vi "SMain.vi"() -> ()   [LabVIEW 2011]
uses:
  Data/ClassLibraryMisWebservice.dll
  dataType/informationIn.ctl
  dataType/singleTestParameter.ctl
  dataType/cluResult.ctl
  dataType/UploadPara.ctl
  Data/Interop.PLTS.dll
  <vilib>/Utility/NIReport.llb/NI_report.lvclass
  dataType/HW_xml.ctl
  Data/xmlFunction.dll
  <vilib>/Utility/file.llb/Read From Spreadsheet File (string).vi
  <vilib>/Utility/file.llb/Write To Spreadsheet File (string).vi
  <vilib>/addons/_office/excel.llb/Excel Easy Table (str).vi
  <vilib>/xml/Load XML File.vi
  <vilib>/regexp/Match Regular Expression.xnode
  <vilib>/Utility/NIReport.llb/Excel/NI_Excel.lvclass
  <vilib>/addons/_office/NI_ReportGenerationToolkit.lvlib
  <vilib>/xml/NI_XML.lvlib
panel:
  out "uploadPara":T1
  out "cluResult":T2
  out "FEXT Results":bool[](array[boolean])
  out "FEXTLIst":string[](array[string])
  out "NEXTList":string[](array[string])
  out "itemList":string[](array[string])
  out "sSpec":T3[](array[typedef])
  out "FEXT INF":T4={"Sample PN: "="", "SampleSN:"="", "Sparam Test Item"=[], "S-para Pair Name"=[], "Length"="", "Diff Test Item Name"=["SDD21", "SDD22", "SCD21", "SCD22", "SCC11", "NEXT", "FEXT"], "Diff Test Item Name smooth"=[], "smooth point"=0.0, "limitSpec"=[], "switchIndexOffset"=0.0, "testType"=enum."Loss"}
  out "NEXT INF":T4={"Sample PN: "="", "SampleSN:"="", "Sparam Test Item"=[], "S-para Pair Name"=[], "Length"="", "Diff Test Item Name"=["SDD21", "SDD22", "SCD21", "SCD22", "SCC11", "NEXT", "FEXT"], "Diff Test Item Name smooth"=[], "smooth point"=0.0, "limitSpec"=[], "switchIndexOffset"=0.0, "testType"=enum."Loss"}
  in  "Information In 2":T4={"Sample PN: "="", "SampleSN:"="", "Sparam Test Item"=[], "S-para Pair Name"=[], "Length"="", "Diff Test Item Name"=["SDD21", "SDD22", "SCD21", "SCD22", "SCC11", "NEXT", "FEXT"], "Diff Test Item Name smooth"=[], "smooth point"=0.0, "limitSpec"=[], "switchIndexOffset"=0.0, "testType"=enum."Loss"}
  out "limitSpec":string[][](array[string])
  in  "Information In":T4={"Sample PN: "="", "SampleSN:"="", "Sparam Test Item"=[], "S-para Pair Name"=[], "Length"="", "Diff Test Item Name"=["SDD21", "SDD22", "SCD21", "SCD22", "SCC11", "NEXT", "FEXT"], "Diff Test Item Name smooth"=[], "smooth point"=0.0, "limitSpec"=[], "switchIndexOffset"=0.0, "testType"=enum."Loss"}
  out "EEUPLOAD":bool
  out "caliData":string
  out "caliPassed":bool
  out "caliDataSelect":bool
  out "sampleData":string
  out "caliFlag":string="cali"
  in  "Stop":bool
  in  "IF Bandwidth:":enum16{"10KHz", "3KHz", "1KHz"}(ring)
  out "FixtureNo":string="111"
  out "LabelNum":i32
  in  "Project Name":u16(ring) items=["QSFP+_10G.xls", "QSFP+_IBM Project.xls"]
  out "S4P Data Path":path=path "D:/高频房软件/2. HPTS_VNA_Rev2.7.1.3-1107最新源码/Demo_data/THRU"
  out "boardCounts":string="Port0 Usage Frequency: 04\nPort1 Usage Frequency: 06" caption="BoardCounts"
  out "preStation":string
  out "original Path":path=path "D:/高频房软件/2. HPTS_VNA_Rev2.7.1.3-1107最新源码/Demo_data"
  in  "Test Spec":u16(ring) items=["EDR_Spec.xls", "QSFP+_10G_IBM.xls"]
  in  "End Page":i32=3
  in  "Start Page":i32=1
  in  "Compensation(ohm)":dbl
  in  "StopTimeNs":dbl=5.0
  in  "Data Points":i32=4000
  in  "Start TimeNs":dbl
  in  "Impedance Filter":bool=TRUE
  in  "Filter Risetime(ps)":dbl=30.0 min=1.0 max=1000.0 step=1.0
  in  "VNA Initial":bool caption="Start Test"
  out "EE Write":bool
  out "正常工单?":bool
  out "PN TYpe":string
  out "PN description":string
  out "NetLocalpath":string
  out "NetTemppath":string
  out "asychronus":bool
  out "show_Cable Point":dbl[](array[numeric])
  out "show_Terminal Point":dbl[](array[numeric])
  out "customerPN":string caption="删减后字符串"
  out "secondresult":bool[](array[boolean])
  out "usedSN":string
  out "Reference":T5
  out "TDR setting array":T6(array[cluster])
  out "CMP setting":string
  out "校验信息":T7(array[cluster])
  out "继续?":bool
  out "DB2":T8
  out "DB1":T8
  out "startSN":i32
  out "线别确认":bool
  out "测试模式":bool
  out "重测原因":string
  out "LastSN":string="automatic sn" caption="S/N:"
  out "TestResultSave":bool
  in  "TestResultSummary":T9={"auto get refer point"=FALSE, "width1"=0, "width2"=0, "show_TDD11"=[], "show_TDD22"=[], "test time"=["2016/11/14 11:59:03"], "show_impspec"=[], "TestResult"=[], "FileName"="", "FileVersion"=""}
  out "TestResult":bool[](array[boolean])
  in  "错误输入（无错误）":errorcluster
  out "2x equalize":bool
  out "Diff Test Item smooth":string[](array[string])=["SDD21", "SDD11,smooth", "SCD22", "SCC11", "SCD21-SDD21", "NEXT", "ILD_15"]
  out "smooth point":i32=5
  out "test result":bool
  out "TDR Setting 2":T10={"Start TimeNs"=0.0, "StopTimeNs"=5.0, "Data Points"=4000, "Compensation(ohm)"=0.0, "DataFormat"=6, "Impedance Filter"=TRUE, "Filter Risetime(ps)"=30.0, "Impedance Spec String"="0.75@110@2@110;0.75@90@2@95", "Skew Spec(ps)"=15, "CMP Setting"=""}
  in  "DataFormat":i16(ring)=6 items=["StepReal", "ImpulseReal", "StepVolts", "ImpulseVolts", "StepLog", "ImpulseLog", "StepImpedance"]
  out "Skew Spec(ps) 2":i32
  out "2X IL 2":dbl[](array[numeric])=[-0.025299, -0.038396, -0.047424, -0.055976, -0.059331, -0.068781, -0.07578, -0.081239, -0.089022, -0.093241, -0.097614, -0.102462, -0.106838, -0.111812, -0.116556, -0.121163, -0.12561, -0.131718, -0.134792, -0.13877, -0.145469, -0.149479, -0.152659, -0.157142, -0.162291, -0.164771, -0.168818, -0.17033, -0.176722, -0.179419, -0.183921, -0.186601, -0.190951, -0.193378, -0.19824, -0.20176, -0.202689, -0.207947, -0.211354, -0.214498, -0.220736, -0.223214, -0.225991, -0.227897, -0.231621, -0.235236, -0.238474, -0.242007, -0.244427, -0.24856, -0.251615, -0.255644, -0.257638, -0.261234, -0.264621, -0.266303, -0.269738, -0.272241, -0.274441, -0.276158, -0.279938, -0.282564, -0.28537, -0.288029, -0.292169, -0.294557, -0.297687, -0.301761, -0.304652, -0.305833, -0.307066, -0.309591, -0.312562, -0.315843, -0.31639, -0.31604, -0.318513, -0.320032, -0.322668, -0.32612, -0.330335, -0.334297, -0.34034, -0.341411, -0.345104, -0.347321, -0.349213, -0.351984, -0.354782, -0.356899, -0.357019, -0.361617, -0.362734, -0.36572, -0.367166, -0.371019, -0.372807, -0.37617, -0.378489, -0.380671, -0.383681, -0.385224, -0.386151, -0.388422, -0.389343, -0.39172, -0.393825, -0.397043, -0.398343, -0.400077, -0.405011, -0.406109, -0.409167, -0.410383, -0.411453, -0.41508, -0.417531, -0.419854, -0.421583, -0.424947, -0.42654, -0.429572, -0.430897, -0.434433, -0.435632, -0.438249, -0.440184, -0.442646, -0.444562, -0.445842, -0.447651, -0.450634, -0.452453, -0.454341, -0.457792, -0.459201, -0.460308, -0.461669, -0.462777, -0.464409, -0.468144, -0.470502, -0.47275, -0.475034, -0.475669, -0.478023, -0.478382, -0.480829, -0.482842, -0.484459, -0.486674, -0.489177, -0.491121, -0.494005, -0.495936, -0.497061, -0.499267, -0.50051, -0.502804, -0.50405, -0.505765, -0.507052, -0.509473, -0.512389, -0.51437, -0.515671, -0.517533, -0.519425, -0.52189, -0.521842, -0.52303, -0.525679, -0.528968, -0.530579, -0.532575, -0.53465, -0.536459, -0.537934, -0.539202, -0.54086, -0.542603, -0.5457, -0.547524, -0.548774, -0.549721, -0.552302, -0.554863, -0.556646, -0.559567, -0.560755, -0.564216, -0.565447, -0.56634, -0.567621, -0.568795, -0.572849, -0.573837, -0.573788, -0.575949, -0.580124, -0.580805, -0.583633, -0.584421, -0.586743, -0.588333, -0.590903, -0.592009, -0.594853, -0.595409, -0.597326, -0.596798, -0.597763, -0.60116, -0.60416, -0.606395, -0.609768, -0.610518, -0.612809, -0.614324, -0.616136, -0.617459, -0.618913, -0.618354, -0.620853, -0.624932, -0.626581, -0.630236, -0.632642, -0.633388, -0.63542, -0.635927, -0.636904, -0.638461, -0.640481, -0.642285, -0.643035, -0.645007, -0.647452, -0.650336, -0.650522, -0.650374, -0.652932, -0.654354, -0.6563, -0.657573, -0.660404, -0.661557, -0.664981, -0.665852, -0.666908, -0.670274, -0.671692, -0.672849, -0.675964, -0.679116, -0.680009, -0.680817, -0.682485, -0.684064, -0.685281, -0.685714, -0.689176, -0.689231, -0.691987, -0.693946, -0.696069, -0.697712, -0.700794, -0.701734, -0.703201, -0.703776, -0.705657, -0.708378, -0.71062, -0.711792, -0.713659, -0.715097, -0.716667, -0.718491, -0.720789, -0.721948, -0.722241, -0.724976, -0.726849, -0.72666, -0.729363, -0.730162, -0.732883, -0.735904, -0.736952, -0.739038, -0.73981, -0.741586, -0.743353, -0.745631, -0.747878, -0.748821, -0.750045, -0.751315, -0.75408, -0.756592, -0.758178, -0.759658, -0.76182, -0.762632, -0.764898, -0.765885, -0.768208, -0.769777, -0.771565, -0.77349, -0.77466, -0.77747, -0.77947, -0.780437, -0.783258, -0.784929, -0.787219, -0.78773, -0.789671, -0.791426, -0.793443, -0.795477, -0.798215, -0.798336, -0.800847, -0.801219, -0.804592, -0.804967, -0.807604, -0.808648, -0.811207, -0.812119, -0.814463, -0.816479, -0.816857, -0.818916, -0.820631, -0.82228, -0.824061, -0.826539, -0.829216, -0.830524, -0.832218, -0.833493, -0.834462, -0.836032, -0.838399, -0.839965, -0.843226, -0.842684, -0.844971, -0.848181, -0.849788, -0.85147, -0.853466, -0.8544, -0.856009, -0.85821, -0.860153, -0.862614, -0.863089, -0.865995, -0.866916, -0.869606, -0.87226, -0.872654, -0.873102, -0.874217, -0.875987, -0.878471, -0.880127, -0.881265, -0.883254, -0.885726, -0.887636, -0.888446, -0.889525, -0.89144, -0.89356, -0.895586, -0.89772, -0.898394, -0.901539, -0.902978, -0.903626, -0.905436, -0.907707, -0.908756, -0.91031, -0.911702, -0.913224, -0.914065, -0.915603, -0.917613, -0.918547, -0.920796, -0.921613, -0.925115, -0.926152, -0.927588, -0.930169, -0.931709, -0.932481, -0.934098, -0.936424, -0.936876, -0.937659, -0.939378, -0.941622, -0.943235, -0.942614, -0.945728, -0.946817, -0.949055, -0.95112, -0.95217, -0.955136, -0.957149, -0.957272, -0.959033, -0.9612, -0.961962, -0.963545, -0.967061, -0.968399, -0.970546, -0.973385, -0.973856, -0.974207, -0.975643, -0.97884, -0.97915, -0.980188, -0.982034, -0.98472, -0.986456, -0.988529, -0.989871, -0.992863, -0.994155, -0.996464, -0.998286, -0.999287, -1.000963, -1.001043, -1.002651, -1.00456, -1.007629, -1.008066, -1.009819, -1.01113, -1.013663, -1.014789, -1.017072, -1.019742, -1.021611, -1.023713, -1.025332, -1.026222, -1.026869, -1.027743, -1.030052, -1.03073, -1.033045, -1.035049, -1.036088, -1.03854, -1.041763, -1.042051, -1.043345, -1.044835, -1.045911, -1.047474, -1.050112, -1.050947, -1.054054, -1.056098, -1.056999, -1.058949, -1.060286, -1.061237, -1.061735, -1.064154, -1.066454, -1.068678, -1.068777, -1.071732, -1.07341, -1.073918, -1.07718, -1.078266, -1.080347, -1.081876, -1.083674, -1.084348, -1.085916, -1.086228, -1.089243, -1.090434, -1.091868, -1.094835, -1.096616, -1.096945, -1.099785, -1.102174, -1.103444, -1.10423, -1.105284, -1.106884, -1.107956, -1.108242, -1.110338, -1.113661, -1.114571, -1.117028, -1.118751, -1.119113, -1.121022, -1.123104, -1.122807, -1.125616, -1.127797, -1.12873, -1.12972, -1.132328, -1.133934, -1.136053, -1.13791, -1.138532, -1.139899, -1.141078, -1.142651, -1.141653, -1.145035, -1.146205, -1.147698, -1.149198, -1.151227, -1.15306, -1.155051, -1.157576, -1.158307, -1.160585, -1.161081, -1.162078, -1.164421, -1.165552, -1.167357, -1.16903, -1.16941, -1.172091, -1.173558, -1.175417, -1.177655, -1.179563, -1.180398, -1.181254, -1.183122, -1.184561, -1.185409, -1.186553, -1.188506, -1.190284, -1.19296, -1.194518, -1.196114, -1.199446, -1.199928, -1.201659, -1.203025, -1.204984, -1.205929, -1.207424, -1.20884, -1.212338, -1.213546, -1.216908, -1.219662, -1.222377, -1.223413, -1.224234, -1.224444, -1.226533, -1.227726, -1.229907, -1.230216, -1.233822, -1.235221, -1.23743, -1.238272, -1.239472, -1.240008, -1.241383, -1.242313, -1.244294, -1.245158, -1.247334, -1.248006, -1.250743, -1.251832, -1.252133, -1.253227, -1.255278, -1.256617, -1.257998, -1.258347, -1.259462, -1.262189, -1.26538, -1.265117, -1.267315, -1.267774, -1.269888, -1.271996, -1.272938, -1.272988, -1.276344, -1.278889, -1.280114, -1.282203, -1.282807, -1.2851, -1.286312, -1.28754, -1.289422, -1.290962, -1.293184, -1.295772, -1.297139, -1.300557, -1.30177, -1.303345, -1.303985, -1.306281, -1.307709, -1.309835, -1.309741, -1.312592, -1.315234, -1.317538, -1.319714, -1.322086, -1.323841, -1.32463, -1.326073, -1.327763, -1.329139, -1.329624, -1.331755, -1.332977, -1.33489, -1.33754, -1.339253, -1.342017, -1.344422, -1.345122, -1.345541, -1.346031, -1.346359, -1.3474, -1.348735, -1.349061, -1.350116, -1.353398, -1.354305, -1.357842, -1.356693, -1.358147, -1.359578, -1.360392, -1.361354, -1.363513, -1.364167, -1.365032, -1.366879, -1.367457, -1.368583, -1.370459, -1.371694, -1.373734, -1.376242, -1.379085, -1.379925, -1.379883, -1.381184, -1.381655, -1.38242, -1.38571, -1.387976, -1.390893, -1.394178, -1.396827, -1.399715, -1.402093, -1.404467, -1.404706, -1.405469, -1.407391, -1.409543, -1.41276, -1.414513, -1.419863, -1.421498, -1.423363, -1.425305, -1.426751, -1.426783, -1.428077, -1.428979, -1.43197, -1.434989, -1.437283, -1.438178, -1.440308, -1.441654, -1.442987, -1.443577, -1.44396, -1.443438, -1.445594, -1.44515, -1.445881, -1.448352, -1.449836, -1.450411, -1.451182, -1.452277, -1.453172, -1.453119, -1.453, -1.453989, -1.456489, -1.456532, -1.458466, -1.458938, -1.460769, -1.462027, -1.462978, -1.462454, -1.464558, -1.46441, -1.466658, -1.466867, -1.468869, -1.47093, -1.472731, -1.47355, -1.474344, -1.474451, -1.476897, -1.478554, -1.479486, -1.481271, -1.483897, -1.484711, -1.487268, -1.488311, -1.489221, -1.49104, -1.491298, -1.491559, -1.493292, -1.496642, -1.497452, -1.499759, -1.501398, -1.502206, -1.506306, -1.506314, -1.508587, -1.509562, -1.51105, -1.511548, -1.514521, -1.516246, -1.518962, -1.522518, -1.52399, -1.526348, -1.526897, -1.529924, -1.531145, -1.532163, -1.533655, -1.534977, -1.536481, -1.538672, -1.541062, -1.542947, -1.544094, -1.543103, -1.545053, -1.546173, -1.547124, -1.548823, -1.550699, -1.552797, -1.552814, -1.553599, -1.555463, -1.557036, -1.556812, -1.559025, -1.557934, -1.559971, -1.563383, -1.565346, -1.567625, -1.568344, -1.569628, -1.571566, -1.571053, -1.572094, -1.571631, -1.575197, -1.576725, -1.579283, -1.580539, -1.582093, -1.583907, -1.58632, -1.587807, -1.589771, -1.590995, -1.591517, -1.593725, -1.595636, -1.596745, -1.596782, -1.598313, -1.601373, -1.600936, -1.602629, -1.605288, -1.606105, -1.608735, -1.609487, -1.612002, -1.612291, -1.612418, -1.615246, -1.612903, -1.614471, -1.615906, -1.618467, -1.619485, -1.621517, -1.623681, -1.626157, -1.6257, -1.627696, -1.629418, -1.631466, -1.632745, -1.633825, -1.636445, -1.639073, -1.640156, -1.642296, -1.642965, -1.644254, -1.646067, -1.645605, -1.647812, -1.648925, -1.650588, -1.653483, -1.654076, -1.655474, -1.656504, -1.659452, -1.660971, -1.661502, -1.661876, -1.66426, -1.665877, -1.665611, -1.668485, -1.66745, -1.668267, -1.668875, -1.670443, -1.671893, -1.673731, -1.676482, -1.677827, -1.679732, -1.68129, -1.681868, -1.684248, -1.687335, -1.689643, -1.691646, -1.693701, -1.696813, -1.699129, -1.699837, -1.700024, -1.702098, -1.704938, -1.708093, -1.709145, -1.712602, -1.715345, -1.717833, -1.720597, -1.721398, -1.723556, -1.72594, -1.726716, -1.726466, -1.72838, -1.729853, -1.729678, -1.731827, -1.734925, -1.738201, -1.741003, -1.742933, -1.742847, -1.743328, -1.743713, -1.745154, -1.746409, -1.748076, -1.74978, -1.750643, -1.754186, -1.754986, -1.756397, -1.758024, -1.758979, -1.759065, -1.760624, -1.760972, -1.762637, -1.761787, -1.763726, -1.765543, -1.765016, -1.766732, -1.766754, -1.767378, -1.769156, -1.770782, -1.769529, -1.771681, -1.774107, -1.774083, -1.773465, -1.776551, -1.7769, -1.777184, -1.779577, -1.782635, -1.784107, -1.784463, -1.785458, -1.788683, -1.788266, -1.788353, -1.792286, -1.794119, -1.797406, -1.799931, -1.799882, -1.803332, -1.805629, -1.808943, -1.810944, -1.815338, -1.817579, -1.821914, -1.823939, -1.823984, -1.824479, -1.827874, -1.828624, -1.831189, -1.834249, -1.837352, -1.840545, -1.842513, -1.843883, -1.844658, -1.845469, -1.847506, -1.847783, -1.847724, -1.849609, -1.851567, -1.854874, -1.855014, -1.856372, -1.857242, -1.857328, -1.857547, -1.857453, -1.856168, -1.857152, -1.858451, -1.860661, -1.863533, -1.862458, -1.862873, -1.8625, -1.864446, -1.864005, -1.865644, -1.867303, -1.869859, -1.869177, -1.87106, -1.872557, -1.87485, -1.876792, -1.87792, -1.879416, -1.880891, -1.88229, -1.883001, -1.884895, -1.887511, -1.888618, -1.889667, -1.890988, -1.89195, -1.893431, -1.894883, -1.897578, -1.898132, -1.900848, -1.902939, -1.903204, -1.906468, -1.907731, -1.911094, -1.914545, -1.914069, -1.916715, -1.919814, -1.924357, -1.925624, -1.926027, -1.927533, -1.92878, -1.930781, -1.933259, -1.935024, -1.935669, -1.937159, -1.941593, -1.943703, -1.944188, -1.94607, -1.94767, -1.949901, -1.953692, -1.956016, -1.95587, -1.956956, -1.957812, -1.960381, -1.959847, -1.962302, -1.964968, -1.965408, -1.966073, -1.966652, -1.968157, -1.96777, -1.968737, -1.969974, -1.971081, -1.973194, -1.973107, -1.973395, -1.975831, -1.974888, -1.976667, -1.977967, -1.979229, -1.978025, -1.979688, -1.981466, -1.982145, -1.98411, -1.985344, -1.987456, -1.986855, -1.98958, -1.991533, -1.99268, -1.994391, -1.995883, -1.998483, -2.001424, -2.002542, -2.003317, -2.005271, -2.005408, -2.007813, -2.010125, -2.014482, -2.01531, -2.017421, -2.019714, -2.020994, -2.022138, -2.024231, -2.024747, -2.027357, -2.029235, -2.029265, -2.030994, -2.031304, -2.034138, -2.036861, -2.040324, -2.041713, -2.042037, -2.04359, -2.044022, -2.044908, -2.046657, -2.047824, -2.051014, -2.054657, -2.056817, -2.059453, -2.061589, -2.06364, -2.065237, -2.067247, -2.068725, -2.071458, -2.074905, -2.07737, -2.080565, -2.083697, -2.087481, -2.091082, -2.092851, -2.093103, -2.093195, -2.093516, -2.095365, -2.096425, -2.099223, -2.101484, -2.103373, -2.105643, -2.106495, -2.106768, -2.106139, -2.107027, -2.108662, -2.110675, -2.113137, -2.114984, -2.114976, -2.114794, -2.115665, -2.115897, -2.116617, -2.115794, -2.118241, -2.118774, -2.119518, -2.120522, -2.120542, -2.123268, -2.121393, -2.122028, -2.122763, -2.123667, -2.125674, -2.126533, -2.126987, -2.127242, -2.129283, -2.130683, -2.133371, -2.134053, -2.135321, -2.136652, -2.137676, -2.1401, -2.141002, -2.144012, -2.146379, -2.149109, -2.149892, -2.151595, -2.153952, -2.157497, -2.159382, -2.16167, -2.163208, -2.164861, -2.164779, -2.165491, -2.168431, -2.171925, -2.177754, -2.178715, -2.183376, -2.185389, -2.186762, -2.190714, -2.190458, -2.191987, -2.195885, -2.198871, -2.204202, -2.207521, -2.209987, -2.21454, -2.218014, -2.21995, -2.220463, -2.220907, -2.221254, -2.22355, -2.225333, -2.229345, -2.23353, -2.235106, -2.238055, -2.24006, -2.240727, -2.239621, -2.236791, -2.239479, -2.238161, -2.241344, -2.245895, -2.245886, -2.247513, -2.250166, -2.250099, -2.250016, -2.248876, -2.248007, -2.247105, -2.247338, -2.249197, -2.249319, -2.250475, -2.25188, -2.251492, -2.252683, -2.252503, -2.251842, -2.251578, -2.250173, -2.252358, -2.254551, -2.255458, -2.258278, -2.258637, -2.259614, -2.262342, -2.263566, -2.265738, -2.267658, -2.271066, -2.275012, -2.277248, -2.281006, -2.283612, -2.285054, -2.287975, -2.292252, -2.296906, -2.299709, -2.304351, -2.306453, -2.30684, -2.31102, -2.313174, -2.316671, -2.31785, -2.319218, -2.323156, -2.326314, -2.329258, -2.331731, -2.330921, -2.335348, -2.337216, -2.338341, -2.339784, -2.341652, -2.345573, -2.345867, -2.348178, -2.350725, -2.350301, -2.348484, -2.346947, -2.348321, -2.34914, -2.350959, -2.353362, -2.356062, -2.357188, -2.36042, -2.360488, -2.359332, -2.359335, -2.35875, -2.358047, -2.358225, -2.358656, -2.359831, -2.358635, -2.360408, -2.360445, -2.361667, -2.361858, -2.362926, -2.363986, -2.364288, -2.36439, -2.366317, -2.367123, -2.367277, -2.367964, -2.370787, -2.371625, -2.372217, -2.375174, -2.376335, -2.378235, -2.380094, -2.383183, -2.385061, -2.386831, -2.391057, -2.392312, -2.396703, -2.400629, -2.403565, -2.406785, -2.410075, -2.412154, -2.414591, -2.416001, -2.418411, -2.421814, -2.426937, -2.431327, -2.43597, -2.438255, -2.439214, -2.441636, -2.442908, -2.443591, -2.444271, -2.446042, -2.447553, -2.451574, -2.454322, -2.459259, -2.459167, -2.458988, -2.459791, -2.459803, -2.460155, -2.460693, -2.460836, -2.461752, -2.464313, -2.467197, -2.467691, -2.467576, -2.466714, -2.466182, -2.465541, -2.466343, -2.466851, -2.466728, -2.468352, -2.469074, -2.468673, -2.470402, -2.472062, -2.472489, -2.4717, -2.474044, -2.476117, -2.475176, -2.475954, -2.477194, -2.478101, -2.478769, -2.482395, -2.482993, -2.485696, -2.489882, -2.491889, -2.493382, -2.4963, -2.497217, -2.495696, -2.497921, -2.498425, -2.499485, -2.502473, -2.505013, -2.507983, -2.511344, -2.514346, -2.515093, -2.515869, -2.515267, -2.517344, -2.516297, -2.517832, -2.521177, -2.524304, -2.525843, -2.529733, -2.532366, -2.533173, -2.533271, -2.533655, -2.534038, -2.534921, -2.537768, -2.538384, -2.540839, -2.543183, -2.545565, -2.547411, -2.547801, -2.550262, -2.549876, -2.551255, -2.551288, -2.55151, -2.55373, -2.556228, -2.55787, -2.560246, -2.561557, -2.56405, -2.564885, -2.56686, -2.568948, -2.568611, -2.571201, -2.573409, -2.574788, -2.577568, -2.579327, -2.581748, -2.583365, -2.586189, -2.588238, -2.588712, -2.5902, -2.592187, -2.593757, -2.594959, -2.595729, -2.597616, -2.599509, -2.602154, -2.604658, -2.607614, -2.60966, -2.610898, -2.61283, -2.613601, -2.613473, -2.613544, -2.616515, -2.620266, -2.623817, -2.625905, -2.631148, -2.636015, -2.640186, -2.641079, -2.645126, -2.645173, -2.647065, -2.649247, -2.651238, -2.654179, -2.659284, -2.66519, -2.667742, -2.672541, -2.674807, -2.673944, -2.674205, -2.673847, -2.674862, -2.67619, -2.680985, -2.685422, -2.6922, -2.698753, -2.698318, -2.697628, -2.696863, -2.697049, -2.696832, -2.697279, -2.698751, -2.702908, -2.706973, -2.710686, -2.713145, -2.713343, -2.712896, -2.71107, -2.708909, -2.707335, -2.707843, -2.70828, -2.711253, -2.71505, -2.720516, -2.723712, -2.725368, -2.726278, -2.724675, -2.72314, -2.723831, -2.722631, -2.724579, -2.727613, -2.731521, -2.734936, -2.739656, -2.743268, -2.746792, -2.750426, -2.752496, -2.755723, -2.757728, -2.759774, -2.761461, -2.765547, -2.772756, -2.77834, -2.784959, -2.791224, -2.797387, -2.800765, -2.804883, -2.808755, -2.808718, -2.813039, -2.817153, -2.823224, -2.831411, -2.838495, -2.843969, -2.849768, -2.853002, -2.856091, -2.857814, -2.858783, -2.860619, -2.865346, -2.870363, -2.877086, -2.88123, -2.886957, -2.887244, -2.886706, -2.885127, -2.880446, -2.879572, -2.879982, -2.883966, -2.885899, -2.890801, -2.894663, -2.892103, -2.888604, -2.88364, -2.878263, -2.874808, -2.869963, -2.868088, -2.86555, -2.867525, -2.869974, -2.86919, -2.870537, -2.869512, -2.866932, -2.865189, -2.861443]
  out "Fix Delay(ns)  2":string="0"
  out "TDR Setting  2":string[](array[string])=["0", "0", "0", "0", "0", "0", "@;@", "0", "0", "-0.025299\t-0.038396\t-0.047424\t-0.055976\t-0.059331\t-0.068781\t-0.075780\t-0.081239\t-0.089022\t-0.093241\t-0.097614\t-0.102462\t-0.106838\t-0.111812\t-0.116556\t-0.121163\t-0.125610\t-0.131718\t-0.134792\t-0.138770\t-0.145469\t-0.149479\t-0.152659\t-0.157142\t-0.162291\t-0.164771\t-0.168818\t-0.170330\t-0.176722\t-0.179419\t-0.183921\t-0.186601\t-0.190951\t-0.193378\t-0.198240\t-0.201760\t-0.202689\t-0.207947\t-0.211354\t-0.214498\t-0.220736\t-0.223214\t-0.225991\t-0.227897\t-0.231621\t-0.235236\t-0.238474\t-0.242007\t-0.244427\t-0.248560\t-0.251615\t-0.255644\t-0.257638\t-0.261234\t-0.264621\t-0.266303\t-0.269738\t-0.272241\t-0.274441\t-0.276158\t-0.279938\t-0.282564\t-0.285370\t-0.288029\t-0.292169\t-0.294557\t-0.297687\t-0.301761\t-0.304652\t-0.305833\t-0.307066\t-0.309591\t-0.312562\t-0.315843\t-0.316390\t-0.316040\t-0.318513\t-0.320032\t-0.322668\t-0.326120\t-0.330335\t-0.334297\t-0.340340\t-0.341411\t-0.345104\t-0.347321\t-0.349213\t-0.351984\t-0.354782\t-0.356899\t-0.357019\t-0.361617\t-0.362734\t-0.365720\t-0.367166\t-0.371019\t-0.372807\t-0.376170\t-0.378489\t-0.380671\t-0.383681\t-0.385224\t-0.386151\t-0.388422\t-0.389343\t-0.391720\t-0.393825\t-0.397043\t-0.398343\t-0.400077\t-0.405011\t-0.406109\t-0.409167\t-0.410383\t-0.411453\t-0.415080\t-0.417531\t-0.419854\t-0.421583\t-0.424947\t-0.426540\t-0.429572\t-0.430897\t-0.434433\t-0.435632\t-0.438249\t-0.440184\t-0.442646\t-0.444562\t-0.445842\t-0.447651\t-0.450634\t-0.452453\t-0.454341\t-0.457792\t-0.459201\t-0.460308\t-0.461669\t-0.462777\t-0.464409\t-0.468144\t-0.470502\t-0.472750\t-0.475034\t-0.475669\t-0.478023\t-0.478382\t-0.480829\t-0.482842\t-0.484459\t-0.486674\t-0.489177\t-0.491121\t-0.494005\t-0.495936\t-0.497061\t-0.499267\t-0.500510\t-0.502804\t-0.504050\t-0.505765\t-0.507052\t-0.509473\t-0.512389\t-0.514370\t-0.515671\t-0.517533\t-0.519425\t-0.521890\t-0.521842\t-0.523030\t-0.525679\t-0.528968\t-0.530579\t-0.532575\t-0.534650\t-0.536459\t-0.537934\t-0.539202\t-0.540860\t-0.542603\t-0.545700\t-0.547524\t-0.548774\t-0.549721\t-0.552302\t-0.554863\t-0.556646\t-0.559567\t-0.560755\t-0.564216\t-0.565447\t-0.566340\t-0.567621\t-0.568795\t-0.572849\t-0.573837\t-0.573788\t-0.575949\t-0.580124\t-0.580805\t-0.583633\t-0.584421\t-0.586743\t-0.588333\t-0.590903\t-0.592009\t-0.594853\t-0.595409\t-0.597326\t-0.596798\t-0.597763\t-0.601160\t-0.604160\t-0.606395\t-0.609768\t-0.610518\t-0.612809\t-0.614324\t-0.616136\t-0.617459\t-0.618913\t-0.618354\t-0.620853\t-0.624932\t-0.626581\t-0.630236\t-0.632642\t-0.633388\t-0.635420\t-0.635927\t-0.636904\t-0.638461\t-0.640481\t-0.642285\t-0.643035\t-0.645007\t-0.647452\t-0.650336\t-0.650522\t-0.650374\t-0.652932\t-0.654354\t-0.656300\t-0.657573\t-0.660404\t-0.661557\t-0.664981\t-0.665852\t-0.666908\t-0.670274\t-0.671692\t-0.672849\t-0.675964\t-0.679116\t-0.680009\t-0.680817\t-0.682485\t-0.684064\t-0.685281\t-0.685714\t-0.689176\t-0.689231\t-0.691987\t-0.693946\t-0.696069\t-0.697712\t-0.700794\t-0.701734\t-0.703201\t-0.703776\t-0.705657\t-0.708378\t-0.710620\t-0.711792\t-0.713659\t-0.715097\t-0.716667\t-0.718491\t-0.720789\t-0.721948\t-0.722241\t-0.724976\t-0.726849\t-0.726660\t-0.729363\t-0.730162\t-0.732883\t-0.735904\t-0.736952\t-0.739038\t-0.739810\t-0.741586\t-0.743353\t-0.745631\t-0.747878\t-0.748821\t-0.750045\t-0.751315\t-0.754080\t-0.756592\t-0.758178\t-0.759658\t-0.761820\t-0.762632\t-0.764898\t-0.765885\t-0.768208\t-0.769777\t-0.771565\t-0.773490\t-0.774660\t-0.777470\t-0.779470\t-0.780437\t-0.783258\t-0.784929\t-0.787219\t-0.787730\t-0.789671\t-0.791426\t-0.793443\t-0.795477\t-0.798215\t-0.798336\t-0.800847\t-0.801219\t-0.804592\t-0.804967\t-0.807604\t-0.808648\t-0.811207\t-0.812119\t-0.814463\t-0.816479\t-0.816857\t-0.818916\t-0.820631\t-0.822280\t-0.824061\t-0.826539\t-0.829216\t-0.830524\t-0.832218\t-0.833493\t-0.834462\t-0.836032\t-0.838399\t-0.839965\t-0.843226\t-0.842684\t-0.844971\t-0.848181\t-0.849788\t-0.851470\t-0.853466\t-0.854400\t-0.856009\t-0.858210\t-0.860153\t-0.862614\t-0.863089\t-0.865995\t-0.866916\t-0.869606\t-0.872260\t-0.872654\t-0.873102\t-0.874217\t-0.875987\t-0.878471\t-0.880127\t-0.881265\t-0.883254\t-0.885726\t-0.887636\t-0.888446\t-0.889525\t-0.891440\t-0.893560\t-0.895586\t-0.897720\t-0.898394\t-0.901539\t-0.902978\t-0.903626\t-0.905436\t-0.907707\t-0.908756\t-0.910310\t-0.911702\t-0.913224\t-0.914065\t-0.915603\t-0.917613\t-0.918547\t-0.920796\t-0.921613\t-0.925115\t-0.926152\t-0.927588\t-0.930169\t-0.931709\t-0.932481\t-0.934098\t-0.936424\t-0.936876\t-0.937659\t-0.939378\t-0.941622\t-0.943235\t-0.942614\t-0.945728\t-0.946817\t-0.949055\t-0.951120\t-0.952170\t-0.955136\t-0.957149\t-0.957272\t-0.959033\t-0.961200\t-0.961962\t-0.963545\t-0.967061\t-0.968399\t-0.970546\t-0.973385\t-0.973856\t-0.974207\t-0.975643\t-0.978840\t-0.979150\t-0.980188\t-0.982034\t-0.984720\t-0.986456\t-0.988529\t-0.989871\t-0.992863\t-0.994155\t-0.996464\t-0.998286\t-0.999287\t-1.000963\t-1.001043\t-1.002651\t-1.004560\t-1.007629\t-1.008066\t-1.009819\t-1.011130\t-1.013663\t-1.014789\t-1.017072\t-1.019742\t-1.021611\t-1.023713\t-1.025332\t-1.026222\t-1.026869\t-1.027743\t-1.030052\t-1.030730\t-1.033045\t-1.035049\t-1.036088\t-1.038540\t-1.041763\t-1.042051\t-1.043345\t-1.044835\t-1.045911\t-1.047474\t-1.050112\t-1.050947\t-1.054054\t-1.056098\t-1.056999\t-1.058949\t-1.060286\t-1.061237\t-1.061735\t-1.064154\t-1.066454\t-1.068678\t-1.068777\t-1.071732\t-1.073410\t-1.073918\t-1.077180\t-1.078266\t-1.080347\t-1.081876\t-1.083674\t-1.084348\t-1.085916\t-1.086228\t-1.089243\t-1.090434\t-1.091868\t-1.094835\t-1.096616\t-1.096945\t-1.099785\t-1.102174\t-1.103444\t-1.104230\t-1.105284\t-1.106884\t-1.107956\t-1.108242\t-1.110338\t-1.113661\t-1.114571\t-1.117028\t-1.118751\t-1.119113\t-1.121022\t-1.123104\t-1.122807\t-1.125616\t-1.127797\t-1.128730\t-1.129720\t-1.132328\t-1.133934\t-1.136053\t-1.137910\t-1.138532\t-1.139899\t-1.141078\t-1.142651\t-1.141653\t-1.145035\t-1.146205\t-1.147698\t-1.149198\t-1.151227\t-1.153060\t-1.155051\t-1.157576\t-1.158307\t-1.160585\t-1.161081\t-1.162078\t-1.164421\t-1.165552\t-1.167357\t-1.169030\t-1.169410\t-1.172091\t-1.173558\t-1.175417\t-1.177655\t-1.179563\t-1.180398\t-1.181254\t-1.183122\t-1.184561\t-1.185409\t-1.186553\t-1.188506\t-1.190284\t-1.192960\t-1.194518\t-1.196114\t-1.199446\t-1.199928\t-1.201659\t-1.203025\t-1.204984\t-1.205929\t-1.207424\t-1.208840\t-1.212338\t-1.213546\t-1.216908\t-1.219662\t-1.222377\t-1.223413\t-1.224234\t-1.224444\t-1.226533\t-1.227726\t-1.229907\t-1.230216\t-1.233822\t-1.235221\t-1.237430\t-1.238272\t-1.239472\t-1.240008\t-1.241383\t-1.242313\t-1.244294\t-1.245158\t-1.247334\t-1.248006\t-1.250743\t-1.251832\t-1.252133\t-1.253227\t-1.255278\t-1.256617\t-1.257998\t-1.258347\t-1.259462\t-1.262189\t-1.265380\t-1.265117\t-1.267315\t-1.267774\t-1.269888\t-1.271996\t-1.272938\t-1.272988\t-1.276344\t-1.278889\t-1.280114\t-1.282203\t-1.282807\t-1.285100\t-1.286312\t-1.287540\t-1.289422\t-1.290962\t-1.293184\t-1.295772\t-1.297139\t-1.300557\t-1.301770\t-1.303345\t-1.303985\t-1.306281\t-1.307709\t-1.309835\t-1.309741\t-1.312592\t-1.315234\t-1.317538\t-1.319714\t-1.322086\t-1.323841\t-1.324630\t-1.326073\t-1.327763\t-1.329139\t-1.329624\t-1.331755\t-1.332977\t-1.334890\t-1.337540\t-1.339253\t-1.342017\t-1.344422\t-1.345122\t-1.345541\t-1.346031\t-1.346359\t-1.347400\t-1.348735\t-1.349061\t-1.350116\t-1.353398\t-1.354305\t-1.357842\t-1.356693\t-1.358147\t-1.359578\t-1.360392\t-1.361354\t-1.363513\t-1.364167\t-1.365032\t-1.366879\t-1.367457\t-1.368583\t-1.370459\t-1.371694\t-1.373734\t-1.376242\t-1.379085\t-1.379925\t-1.379883\t-1.381184\t-1.381655\t-1.382420\t-1.385710\t-1.387976\t-1.390893\t-1.394178\t-1.396827\t-1.399715\t-1.402093\t-1.404467\t-1.404706\t-1.405469\t-1.407391\t-1.409543\t-1.412760\t-1.414513\t-1.419863\t-1.421498\t-1.423363\t-1.425305\t-1.426751\t-1.426783\t-1.428077\t-1.428979\t-1.431970\t-1.434989\t-1.437283\t-1.438178\t-1.440308\t-1.441654\t-1.442987\t-1.443577\t-1.443960\t-1.443438\t-1.445594\t-1.445150\t-1.445881\t-1.448352\t-1.449836\t-1.450411\t-1.451182\t-1.452277\t-1.453172\t-1.453119\t-1.453000\t-1.453989\t-1.456489\t-1.456532\t-1.458466\t-1.458938\t-1.460769\t-1.462027\t-1.462978\t-1.462454\t-1.464558\t-1.464410\t-1.466658\t-1.466867\t-1.468869\t-1.470930\t-1.472731\t-1.473550\t-1.474344\t-1.474451\t-1.476897\t-1.478554\t-1.479486\t-1.481271\t-1.483897\t-1.484711\t-1.487268\t-1.488311\t-1.489221\t-1.491040\t-1.491298\t-1.491559\t-1.493292\t-1.496642\t-1.497452\t-1.499759\t-1.501398\t-1.502206\t-1.506306\t-1.506314\t-1.508587\t-1.509562\t-1.511050\t-1.511548\t-1.514521\t-1.516246\t-1.518962\t-1.522518\t-1.523990\t-1.526348\t-1.526897\t-1.529924\t-1.531145\t-1.532163\t-1.533655\t-1.534977\t-1.536481\t-1.538672\t-1.541062\t-1.542947\t-1.544094\t-1.543103\t-1.545053\t-1.546173\t-1.547124\t-1.548823\t-1.550699\t-1.552797\t-1.552814\t-1.553599\t-1.555463\t-1.557036\t-1.556812\t-1.559025\t-1.557934\t-1.559971\t-1.563383\t-1.565346\t-1.567625\t-1.568344\t-1.569628\t-1.571566\t-1.571053\t-1.572094\t-1.571631\t-1.575197\t-1.576725\t-1.579283\t-1.580539\t-1.582093\t-1.583907\t-1.586320\t-1.587807\t-1.589771\t-1.590995\t-1.591517\t-1.593725\t-1.595636\t-1.596745\t-1.596782\t-1.598313\t-1.601373\t-1.600936\t-1.602629\t-1.605288\t-1.606105\t-1.608735\t-1.609487\t-1.612002\t-1.612291\t-1.612418\t-1.615246\t-1.612903\t-1.614471\t-1.615906\t-1.618467\t-1.619485\t-1.621517\t-1.623681\t-1.626157\t-1.625700\t-1.627696\t-1.629418\t-1.631466\t-1.632745\t-1.633825\t-1.636445\t-1.639073\t-1.640156\t-1.642296\t-1.642965\t-1.644254\t-1.646067\t-1.645605\t-1.647812\t-1.648925\t-1.650588\t-1.653483\t-1.654076\t-1.655474\t-1.656504\t-1.659452\t-1.660971\t-1.661502\t-1.661876\t-1.664260\t-1.665877\t-1.665611\t-1.668485\t-1.667450\t-1.668267\t-1.668875\t-1.670443\t-1.671893\t-1.673731\t-1.676482\t-1.677827\t-1.679732\t-1.681290\t-1.681868\t-1.684248\t-1.687335\t-1.689643\t-1.691646\t-1.693701\t-1.696813\t-1.699129\t-1.699837\t-1.700024\t-1.702098\t-1.704938\t-1.708093\t-1.709145\t-1.712602\t-1.715345\t-1.717833\t-1.720597\t-1.721398\t-1.723556\t-1.725940\t-1.726716\t-1.726466\t-1.728380\t-1.729853\t-1.729678\t-1.731827\t-1.734925\t-1.738201\t-1.741003\t-1.742933\t-1.742847\t-1.743328\t-1.743713\t-1.745154\t-1.746409\t-1.748076\t-1.749780\t-1.750643\t-1.754186\t-1.754986\t-1.756397\t-1.758024\t-1.758979\t-1.759065\t-1.760624\t-1.760972\t-1.762637\t-1.761787\t-1.763726\t-1.765543\t-1.765016\t-1.766732\t-1.766754\t-1.767378\t-1.769156\t-1.770782\t-1.769529\t-1.771681\t-1.774107\t-1.774083\t-1.773465\t-1.776551\t-1.776900\t-1.777184\t-1.779577\t-1.782635\t-1.784107\t-1.784463\t-1.785458\t-1.788683\t-1.788266\t-1.788353\t-1.792286\t-1.794119\t-1.797406\t-1.799931\t-1.799882\t-1.803332\t-1.805629\t-1.808943\t-1.810944\t-1.815338\t-1.817579\t-1.821914\t-1.823939\t-1.823984\t-1.824479\t-1.827874\t-1.828624\t-1.831189\t-1.834249\t-1.837352\t-1.840545\t-1.842513\t-1.843883\t-1.844658\t-1.845469\t-1.847506\t-1.847783\t-1.847724\t-1.849609\t-1.851567\t-1.854874\t-1.855014\t-1.856372\t-1.857242\t-1.857328\t-1.857547\t-1.857453\t-1.856168\t-1.857152\t-1.858451\t-1.860661\t-1.863533\t-1.862458\t-1.862873\t-1.862500\t-1.864446\t-1.864005\t-1.865644\t-1.867303\t-1.869859\t-1.869177\t-1.871060\t-1.872557\t-1.874850\t-1.876792\t-1.877920\t-1.879416\t-1.880891\t-1.882290\t-1.883001\t-1.884895\t-1.887511\t-1.888618\t-1.889667\t-1.890988\t-1.891950\t-1.893431\t-1.894883\t-1.897578\t-1.898132\t-1.900848\t-1.902939\t-1.903204\t-1.906468\t-1.907731\t-1.911094\t-1.914545\t-1.914069\t-1.916715\t-1.919814\t-1.924357\t-1.925624\t-1.926027\t-1.927533\t-1.928780\t-1.930781\t-1.933259\t-1.935024\t-1.935669\t-1.937159\t-1.941593\t-1.943703\t-1.944188\t-1.946070\t-1.947670\t-1.949901\t-1.953692\t-1.956016\t-1.955870\t-1.956956\t-1.957812\t-1.960381\t-1.959847\t-1.962302\t-1.964968\t-1.965408\t-1.966073\t-1.966652\t-1.968157\t-1.967770\t-1.968737\t-1.969974\t-1.971081\t-1.973194\t-1.973107\t-1.973395\t-1.975831\t-1.974888\t-1.976667\t-1.977967\t-1.979229\t-1.978025\t-1.979688\t-1.981466\t-1.982145\t-1.984110\t-1.985344\t-1.987456\t-1.986855\t-1.989580\t-1.991533\t-1.992680\t-1.994391\t-1.995883\t-1.998483\t-2.001424\t-2.002542\t-2.003317\t-2.005271\t-2.005408\t-2.007813\t-2.010125\t-2.014482\t-2.015310\t-2.017421\t-2.019714\t-2.020994\t-2.022138\t-2.024231\t-2.024747\t-2.027357\t-2.029235\t-2.029265\t-2.030994\t-2.031304\t-2.034138\t-2.036861\t-2.040324\t-2.041713\t-2.042037\t-2.043590\t-2.044022\t-2.044908\t-2.046657\t-2.047824\t-2.051014\t-2.054657\t-2.056817\t-2.059453\t-2.061589\t-2.063640\t-2.065237\t-2.067247\t-2.068725\t-2.071458\t-2.074905\t-2.077370\t-2.080565\t-2.083697\t-2.087481\t-2.091082\t-2.092851\t-2.093103\t-2.093195\t-2.093516\t-2.095365\t-2.096425\t-2.099223\t-2.101484\t-2.103373\t-2.105643\t-2.106495\t-2.106768\t-2.106139\t-2.107027\t-2.108662\t-2.110675\t-2.113137\t-2.114984\t-2.114976\t-2.114794\t-2.115665\t-2.115897\t-2.116617\t-2.115794\t-2.118241\t-2.118774\t-2.119518\t-2.120522\t-2.120542\t-2.123268\t-2.121393\t-2.122028\t-2.122763\t-2.123667\t-2.125674\t-2.126533\t-2.126987\t-2.127242\t-2.129283\t-2.130683\t-2.133371\t-2.134053\t-2.135321\t-2.136652\t-2.137676\t-2.140100\t-2.141002\t-2.144012\t-2.146379\t-2.149109\t-2.149892\t-2.151595\t-2.153952\t-2.157497\t-2.159382\t-2.161670\t-2.163208\t-2.164861\t-2.164779\t-2.165491\t-2.168431\t-2.171925\t-2.177754\t-2.178715\t-2.183376\t-2.185389\t-2.186762\t-2.190714\t-2.190458\t-2.191987\t-2.195885\t-2.198871\t-2.204202\t-2.207521\t-2.209987\t-2.214540\t-2.218014\t-2.219950\t-2.220463\t-2.220907\t-2.221254\t-2.223550\t-2.225333\t-2.229345\t-2.233530\t-2.235106\t-2.238055\t-2.240060\t-2.240727\t-2.239621\t-2.236791\t-2.239479\t-2.238161\t-2.241344\t-2.245895\t-2.245886\t-2.247513\t-2.250166\t-2.250099\t-2.250016\t-2.248876\t-2.248007\t-2.247105\t-2.247338\t-2.249197\t-2.249319\t-2.250475\t-2.251880\t-2.251492\t-2.252683\t-2.252503\t-2.251842\t-2.251578\t-2.250173\t-2.252358\t-2.254551\t-2.255458\t-2.258278\t-2.258637\t-2.259614\t-2.262342\t-2.263566\t-2.265738\t-2.267658\t-2.271066\t-2.275012\t-2.277248\t-2.281006\t-2.283612\t-2.285054\t-2.287975\t-2.292252\t-2.296906\t-2.299709\t-2.304351\t-2.306453\t-2.306840\t-2.311020\t-2.313174\t-2.316671\t-2.317850\t-2.319218\t-2.323156\t-2.326314\t-2.329258\t-2.331731\t-2.330921\t-2.335348\t-2.337216\t-2.338341\t-2.339784\t-2.341652\t-2.345573\t-2.345867\t-2.348178\t-2.350725\t-2.350301\t-2.348484\t-2.346947\t-2.348321\t-2.349140\t-2.350959\t-2.353362\t-2.356062\t-2.357188\t-2.360420\t-2.360488\t-2.359332\t-2.359335\t-2.358750\t-2.358047\t-2.358225\t-2.358656\t-2.359831\t-2.358635\t-2.360408\t-2.360445\t-2.361667\t-2.361858\t-2.362926\t-2.363986\t-2.364288\t-2.364390\t-2.366317\t-2.367123\t-2.367277\t-2.367964\t-2.370787\t-2.371625\t-2.372217\t-2.375174\t-2.376335\t-2.378235\t-2.380094\t-2.383183\t-2.385061\t-2.386831\t-2.391057\t-2.392312\t-2.396703\t-2.400629\t-2.403565\t-2.406785\t-2.410075\t-2.412154\t-2.414591\t-2.416001\t-2.418411\t-2.421814\t-2.426937\t-2.431327\t-2.435970\t-2.438255\t-2.439214\t-2.441636\t-2.442908\t-2.443591\t-2.444271\t-2.446042\t-2.447553\t-2.451574\t-2.454322\t-2.459259\t-2.459167\t-2.458988\t-2.459791\t-2.459803\t-2.460155\t-2.460693\t-2.460836\t-2.461752\t-2.464313\t-2.467197\t-2.467691\t-2.467576\t-2.466714\t-2.466182\t-2.465541\t-2.466343\t-2.466851\t-2.466728\t-2.468352\t-2.469074\t-2.468673\t-2.470402\t-2.472062\t-2.472489\t-2.471700\t-2.474044\t-2.476117\t-2.475176\t-2.475954\t-2.477194\t-2.478101\t-2.478769\t-2.482395\t-2.482993\t-2.485696\t-2.489882\t-2.491889\t-2.493382\t-2.496300\t-2.497217\t-2.495696\t-2.497921\t-2.498425\t-2.499485\t-2.502473\t-2.505013\t-2.507983\t-2.511344\t-2.514346\t-2.515093\t-2.515869\t-2.515267\t-2.517344\t-2.516297\t-2.517832\t-2.521177\t-2.524304\t-2.525843\t-2.529733\t-2.532366\t-2.533173\t-2.533271\t-2.533655\t-2.534038\t-2.534921\t-2.537768\t-2.538384\t-2.540839\t-2.543183\t-2.545565\t-2.547411\t-2.547801\t-2.550262\t-2.549876\t-2.551255\t-2.551288\t-2.551510\t-2.553730\t-2.556228\t-2.557870\t-2.560246\t-2.561557\t-2.564050\t-2.564885\t-2.566860\t-2.568948\t-2.568611\t-2.571201\t-2.573409\t-2.574788\t-2.577568\t-2.579327\t-2.581748\t-2.583365\t-2.586189\t-2.588238\t-2.588712\t-2.590200\t-2.592187\t-2.593757\t-2.594959\t-2.595729\t-2.597616\t-2.599509\t-2.602154\t-2.604658\t-2.607614\t-2.609660\t-2.610898\t-2.612830\t-2.613601\t-2.613473\t-2.613544\t-2.616515\t-2.620266\t-2.623817\t-2.625905\t-2.631148\t-2.636015\t-2.640186\t-2.641079\t-2.645126\t-2.645173\t-2.647065\t-2.649247\t-2.651238\t-2.654179\t-2.659284\t-2.665190\t-2.667742\t-2.672541\t-2.674807\t-2.673944\t-2.674205\t-2.673847\t-2.674862\t-2.676190\t-2.680985\t-2.685422\t-2.692200\t-2.698753\t-2.698318\t-2.697628\t-2.696863\t-2.697049\t-2.696832\t-2.697279\t-2.698751\t-2.702908\t-2.706973\t-2.710686\t-2.713145\t-2.713343\t-2.712896\t-2.711070\t-2.708909\t-2.707335\t-2.707843\t-2.708280\t-2.711253\t-2.715050\t-2.720516\t-2.723712\t-2.725368\t-2.726278\t-2.724675\t-2.723140\t-2.723831\t-2.722631\t-2.724579\t-2.727613\t-2.731521\t-2.734936\t-2.739656\t-2.743268\t-2.746792\t-2.750426\t-2.752496\t-2.755723\t-2.757728\t-2.759774\t-2.761461\t-2.765547\t-2.772756\t-2.778340\t-2.784959\t-2.791224\t-2.797387\t-2.800765\t-2.804883\t-2.808755\t-2.808718\t-2.813039\t-2.817153\t-2.823224\t-2.831411\t-2.838495\t-2.843969\t-2.849768\t-2.853002\t-2.856091\t-2.857814\t-2.858783\t-2.860619\t-2.865346\t-2.870363\t-2.877086\t-2.881230\t-2.886957\t-2.887244\t-2.886706\t-2.885127\t-2.880446\t-2.879572\t-2.879982\t-2.883966\t-2.885899\t-2.890801\t-2.894663\t-2.892103\t-2.888604\t-2.883640\t-2.878263\t-2.874808\t-2.869963\t-2.868088\t-2.865550\t-2.867525\t-2.869974\t-2.869190\t-2.870537\t-2.869512\t-2.866932\t-2.865189\t-2.861443"]
  in  "Impedance Spec String 2":string="@;@"
  in  "Data Points 2":i32
  in  "Compensation(ohm) 2":dbl
  in  "StopTimeNs 2":dbl
  in  "Start TimeNs 2":dbl
  in  "Impedance Filter 2":bool
  in  "Filter Risetime(ps) 2":dbl min=1.0 max=1000.0 step=1.0
  out "width2":i32
  out "width1":i32
  out "auto get refer point":bool
  out "SystemMode":string="GPF001"
  out "Count":i16=1
  out "DateCode8Value_0X30":i32=32 format="%x"
  out "ConvertStyle":bool
  out "CountXmlPath":path=path "D:/高频房软件/2. HPTS_VNA_Rev2.7.1.3-1107最新源码/DataBase/L99QF015-SD-R/20161114.xml"
  out "PassCount?":bool=TRUE
  out "upload":bool
  out "AlarmDisplay":bool=TRUE
  out "NetPathCompress2":path=path "\\\\172.20.20.113\\emc/HPTS/SI"
  out "NetPathCompress1":path=path "\\\\172.20.20.113\\emc/HPTS/VNA"
  out "NetCmdCompress":string="net use \\\\172.20.20.113 mesuser /user:mesuser"
  out "NetPathHW":string="\\\\172.20.20.86\\HuaweiData\\DataRoot\\XML"
  out "NetCmd":string="net use \\\\172.20.20.86 Luxshare-ict /user:C040345"
  out "NEXTList":string[](array[string])=["TX1-RX1", "TX2-RX1", "TX3-RX1", "TX4-RX1", "TX1-RX2", "TX2-RX2", "TX3-RX2", "TX4-RX2", "TX1-RX3", "TX2-RX3", "TX3-RX3", "TX4-RX3", "TX1-RX4", "TX2-RX4", "TX3-RX4", "TX4-RX4"]
  out "NEXTReults":bool[](array[boolean])
  out "SparaLists":string[](array[string])=["SDD21", "SDD11", "SCD22", "SCC11", "SCD21-SDD21", "ILD_15", "TDD11", "TDD22", "Pskew"]
  out "SparaReults":bool[](array[boolean])=[FALSE, FALSE, FALSE, FALSE, FALSE, TRUE, FALSE, FALSE, TRUE]
  out "FullXml":bool
  out "CustomerName":string="HuaWei"
  out "FileName":string="DevelopmentSystem"
  out "FileVersion":string="DevelopmentSystem"
  out "S写入延时（单位：ms） 2":dbl
  out "读取延时（单位：ms） 2":dbl
  out "Q写入延时（单位：ms） 2":dbl
  out "Test Status: 2":string="\n当前datacode为:0X20\n自动生成序列号小于本地MDB数据库记录SN，系统天数=数据库记录天数，生成流水号从数据库\n历史记录+1\nStart Test at 周一 上午 11:24:03 2016/11/14 China Time On wmg-PC.luxshare.com.cn\rP/N:L99QF015-SD-R,  Sample S/N:201611145014,  Length:1000mm\rThe Test Is Performed In Accordance With Related SI Spec\rS-parameter Testing.....\rSDD21_TX1:NG\rSDD11_TX1:NG\rSCD22_TX1:NG\rSCC11_TX1:NG\rSCD21-SDD21_TX1:NG\rTDD11_TX1:NG\rMax 133.38 117.59 \rMin 111.42 114.43 \rTDD22_TX1:NG\rMax 133.03 116.62 \rMin 109.85 113.82 \rTX1_Intra-pair Skew:0ps,OK (Spec max:15ps)\rSDD21_RX1:NG\rSDD11_RX1:NG\rSCD22_RX1:NG\rSCC11_RX1:NG\rSCD21-SDD21_RX1:NG\rTDD11_RX1:NG\rMax 128.10 116.52 \rMin 111.49 111.54 \rTDD22_RX1:NG\rMax 128.33 114.73 \rMin 108.98 109.00 \rRX1_Intra-pair Skew:0ps,OK (Spec max:15ps)\rSDD21_TX2:NG\rSDD11_TX2:NG\rSCD22_TX2:NG\rSCC11_TX2:NG\rSCD21-SDD21_TX2:NG\rTDD11_TX2:NG\rMax 129.55 115.75 \rMin 110.56 114.32 \rTDD22_TX2:NG\rMax 129.05 116.28 \rMin 108.99 114.50 \rTX2_Intra-pair Skew:0ps,OK (Spec max:15ps)\rSDD21_RX2:NG\rSDD11_RX2:NG\rSCD22_RX2:NG\rSCC11_RX2:NG\rSCD21-SDD21_RX2:NG\rTDD11_RX2:NG\rMax 129.31 117.05 \rMin 110.95 115.67 \rTDD22_RX2:NG\rMax 128.69 115.98 \rMin 110.50 114.65 \rRX2_Intra-pair Skew:0ps,OK (Spec max:15ps)\rSDD21_TX3:NG\rSDD11_TX3:NG\rSCD22_TX3:NG\rSCC11_TX3:NG\rSCD21-SDD21_TX3:NG\rTDD22_TX3:NG\rMax 133.03 114.43 \rMin 104.67 113.35 \rTDD11_TX3:NG\rMax 132.35 116.87 \rMin 104.39 115.18 \rTX3_Intra-pair Skew:0ps,OK (Spec max:15ps)\rSDD21_RX3:NG\rSDD11_RX3:NG\rSCD22_RX3:NG\rSCC11_RX3:NG\rSCD21-SDD21_RX3:NG\rTDD22_RX3:NG\rMax 127.53 115.30 \rMin 111.10 114.17 \rTDD11_RX3:NG\rMax 128.36 113.46 \rMin 109.35 111.72 \rRX3_Intra-pair Skew:0ps,OK (Spec max:15ps)\rSDD21_TX4:NG\rSDD11_TX4:NG\rSCD22_TX4:NG\rSCC11_TX4:NG\rSCD21-SDD21_TX4:NG\rTDD22_TX4:NG\rMax 128.13 114.91 \rMin 112.44 113.68 \rTDD11_TX4:NG\rMax 129.10 115.37 \rMin 111.66 113.97 \rTX4_Intra-pair Skew:0ps,OK (Spec max:15ps)\rSDD21_RX4:NG\rSDD11_RX4:NG\rSCD22_RX4:OK\rSCC11_RX4:NG\rSCD21-SDD21_RX4:NG\rTDD22_RX4:NG\rMax 133.06 117.74 \rMin 103.32 115.49 \rTDD11_RX4:NG\rMax 132.17 116.99 \rMin 102.07 114.63 \rRX4_Intra-pair Skew:0ps,OK (Spec max:15ps)\rSDD21_Total_Result:Fail\rSDD11_Total_Result:Fail\rSCD22_Total_Result:Fail\rSCC11_Total_Result:Fail\rSCD21-SDD21_Total_Result:Fail\rILD_15_Total_Result:Pass\rTDD11_Total_Result:Fail\rTDD22_Total_Result:Fail\rPskew_Total_Result:Pass\nWrite EEprom\nRead EEprom\nPort 0: FAIL\nPort 1: FAIL\nDemo mode Label has been printed!\n201611145014 :Test Finished !\rEnded Test At 周一 上午 11:25:36 2016/11/14 China Time.  Test Time: 93.165329s"
  out "未经进制转换的sn(客户 jin zhi sn)":string
  out "Shi jin zhi sn":string
  out "customer date":string
  out "S写入延时（单位：ms）":dbl=100.0
  out "读取延时（单位：ms）":dbl=100.0
  out "Q写入延时（单位：ms）":dbl=250.0
  out "要烧录的DateCode":string
  out "要烧录的时间和Sn":string
  out "result":bool=TRUE
  out "Data Out  2":u8[](array[numeric])=[0, 4, 0, 16]
  out "无符号字节数组":u8[](array[numeric])=[238, 0, 17, 0, 0, 128, 0, 4, 0, 4, 0, 16, 129, 255, 252, 255, 255] format="%.0x"
  out "strFSN 原始SN":string
  out "PRINT":refnum<k24>
  out "SN":refnum<k24>
  in  "labelConfig":string[](array[string])=["年周", "17", "18", "", "", "19", "20", "22", "22", "23", "27", "Z00A2Ryyww(X6)", "", "", "1", "0", ""]
  out "Go":bool
  out "cableType":string
  out "mid_str_descrip":string="年周"
  out "mid_array_temp_int":u8[][](array[numeric])=[[17, 6, 6, 0, 0, 0, 0, 0, 0, 0, 0, 0, 0, 0, 0, 0, 0, 0, 0, 0, 0, 0, 0, 0, 0, 0, 0, 0, 0, 0, 0, 0, 0, 0, 0, 0, 0, 0, 0, 0, 0, 0, 0, 0, 0, 0, 0, 0, 0, 0, 0, 0, 0, 0, 0, 0, 0, 0, 0, 0, 0, 0, 0, 0, 0, 0, 0, 0, 0, 0, 0, 0, 0, 0, 0, 0, 0, 0, 0, 0, 0, 0, 0, 0, 0, 0, 0, 0, 0, 0, 0, 0, 0, 0, 0, 0, 0, 0, 0, 0, 0, 0, 0, 0, 0, 0, 0, 0, 0, 0, 56, 0, 0, 0, 0, 0, 0, 0, 0, 0, 0, 0, 0, 0, 0, 0, 0, 0, 17, 0, 35, 136, 0, 0, 0, 0, 0, 128, 0, 5, 255, 0, 0, 0, 0, 0, 1, 160, 76, 85, 88, 83, 72, 65, 82, 69, 45, 73, 67, 84, 32, 32, 32, 32, 31, 60, 24, 160, 76, 57, 57, 81, 70, 48, 49, 53, 45, 83, 68, 45, 82, 32, 32, 32, 66, 32, 3, 4, 5, 8, 70, 55, 11, 0, 0, 0, 90, 48, 48, 65, 50, 82, 49, 54, 52, 55, 48, 48, 53, 48, 49, 56, 49, 54, 49, 49, 49, 52, 32, 32, 0, 0, 103, 95, 0, 0, 0, 0, 0, 0, 0, 0, 0, 0, 0, 0, 0, 0, 0, 0, 0, 0, 0, 0, 0, 0, 0, 0, 0, 0, 0, 0, 0, 0, 0, 0], [17, 6, 6, 0, 0, 0, 0, 0, 0, 0, 0, 0, 0, 0, 0, 0, 0, 0, 0, 0, 0, 0, 0, 0, 0, 0, 0, 0, 0, 0, 0, 0, 0, 0, 0, 0, 0, 0, 0, 0, 0, 0, 0, 0, 0, 0, 0, 0, 0, 0, 0, 0, 0, 0, 0, 0, 0, 0, 0, 0, 0, 0, 0, 0, 0, 0, 0, 0, 0, 0, 0, 0, 0, 0, 0, 0, 0, 0, 0, 0, 0, 0, 0, 0, 0, 0, 0, 0, 0, 0, 0, 0, 0, 0, 0, 0, 0, 0, 0, 0, 0, 0, 0, 0, 0, 0, 0, 0, 0, 0, 56, 0, 0, 0, 0, 0, 0, 0, 0, 0, 0, 0, 0, 0, 0, 0, 0, 0, 17, 0, 35, 136, 0, 0, 0, 0, 0, 128, 0, 5, 255, 0, 0, 0, 0, 0, 1, 160, 76, 85, 88, 83, 72, 65, 82, 69, 45, 73, 67, 84, 32, 32, 32, 32, 31, 60, 24, 160, 76, 57, 57, 81, 70, 48, 49, 53, 45, 83, 68, 45, 82, 32, 32, 32, 66, 32, 3, 4, 5, 8, 70, 55, 11, 0, 0, 0, 90, 48, 48, 65, 50, 82, 49, 54, 52, 55, 48, 48, 53, 48, 49, 56, 49, 54, 49, 49, 49, 52, 32, 32, 0, 0, 103, 95, 0, 0, 0, 0, 0, 0, 0, 0, 0, 0, 0, 0, 0, 0, 0, 0, 0, 0, 0, 0, 0, 0, 0, 0, 0, 0, 0, 0, 0, 0, 0, 0]] format="%.0x"
  out "mid_str_snformat":string="Z00A2Ryyww(X6)"
  out "mid_str_labelType":string="QSFP+28_HW"
  out "mid_array_eep":string[][](array[string])=[["11", "11"], ["6", "6"], ["6", "6"], ["0", "0"], ["0", "0"], ["0", "0"], ["0", "0"], ["0", "0"], ["0", "0"], ["0", "0"], ["0", "0"], ["0", "0"], ["0", "0"], ["0", "0"], ["0", "0"], ["0", "0"], ["0", "0"], ["0", "0"], ["0", "0"], ["0", "0"], ["0", "0"], ["0", "0"], ["0", "0"], ["0", "0"], ["0", "0"], ["0", "0"], ["0", "0"], ["0", "0"], ["0", "0"], ["0", "0"], ["0", "0"], ["0", "0"], ["0", "0"], ["0", "0"], ["0", "0"], ["0", "0"], ["0", "0"], ["0", "0"], ["0", "0"], ["0", "0"], ["0", "0"], ["0", "0"], ["0", "0"], ["0", "0"], ["0", "0"], ["0", "0"], ["0", "0"], ["0", "0"], ["0", "0"], ["0", "0"], ["0", "0"], ["0", "0"], ["0", "0"], ["0", "0"], ["0", "0"], ["0", "0"], ["0", "0"], ["0", "0"], ["0", "0"], ["0", "0"], ["0", "0"], ["0", "0"], ["0", "0"], ["0", "0"], ["0", "0"], ["0", "0"], ["0", "0"], ["0", "0"], ["0", "0"], ["0", "0"], ["0", "0"], ["0", "0"], ["0", "0"], ["0", "0"], ["0", "0"], ["0", "0"], ["0", "0"], ["0", "0"], ["0", "0"], ["0", "0"], ["0", "0"], ["0", "0"], ["0", "0"], ["0", "0"], ["0", "0"], ["0", "0"], ["0", "0"], ["0", "0"], ["0", "0"], ["0", "0"], ["0", "0"], ["0", "0"], ["0", "0"], ["0", "0"], ["0", "0"], ["0", "0"], ["0", "0"], ["0", "0"], ["0", "0"], ["0", "0"], ["0", "0"], ["0", "0"], ["0", "0"], ["0", "0"], ["0", "0"], ["0", "0"], ["0", "0"], ["0", "0"], ["0", "0"], ["0", "0"], ["38", "38"], ["0", "0"], ["0", "0"], ["0", "0"], ["0", "0"], ["0", "0"], ["0", "0"], ["0", "0"], ["0", "0"], ["0", "0"], ["0", "0"], ["0", "0"], ["0", "0"], ["0", "0"], ["0", "0"], ["0", "0"], ["0", "0"], ["0", "0"], ["11", "11"], ["0", "0"], ["23", "23"], ["88", "88"], ["0", "0"], ["0", "0"], ["0", "0"], ["0", "0"], ["0", "0"], ["80", "80"], ["0", "0"], ["5", "5"], ["FF", "FF"], ["0", "0"], ["0", "0"], ["0", "0"], ["0", "0"], ["0", "0"], ["1", "1"], ["A0", "A0"], ["4C", "4C"], ["55", "55"], ["58", "58"], ["53", "53"], ["48", "48"], ["41", "41"], ["52", "52"], ["45", "45"], ["2D", "2D"], ["49", "49"], ["43", "43"], ["54", "54"], ["20", "20"], ["20", "20"], ["20", "20"], ["20", "20"], ["1F", "1F"], ["3C", "3C"], ["18", "18"], ["A0", "A0"], ["4C", "4C"], ["39", "39"], ["39", "39"], ["51", "51"], ["46", "46"], ["30", "30"], ["31", "31"], ["35", "35"], ["2D", "2D"], ["53", "53"], ["44", "44"], ["2D", "2D"], ["52", "52"], ["20", "20"], ["20", "20"], ["20", "20"], ["42", "42"], ["20", "20"], ["3", "3"], ["4", "4"], ["5", "5"], ["8", "8"], ["46", "46"], ["0", "0"], ["0B", "0B"], ["0", "0"], ["0", "0"], ["0", "0"], ["5A", "5A"], ["30", "30"], ["30", "30"], ["41", "41"], ["32", "32"], ["52", "52"], ["20", "20"], ["20", "20"], ["20", "20"], ["20", "20"], ["20", "20"], ["20", "20"], ["20", "20"], ["20", "20"], ["20", "20"], ["20", "20"], ["20", "20"], ["20", "20"], ["20", "20"], ["20", "20"], ["20", "20"], ["20", "20"], ["20", "20"], ["20", "20"], ["0", "0"], ["0", "0"], ["67", "67"], ["0", "0"], ["0", "0"], ["0", "0"], ["0", "0"], ["0", "0"], ["0", "0"], ["0", "0"], ["0", "0"], ["0", "0"], ["0", "0"], ["0", "0"], ["0", "0"], ["0", "0"], ["0", "0"], ["0", "0"], ["0", "0"], ["0", "0"], ["0", "0"], ["0", "0"], ["0", "0"], ["0", "0"], ["0", "0"], ["0", "0"], ["0", "0"], ["0", "0"], ["0", "0"], ["0", "0"], ["0", "0"], ["0", "0"], ["0", "0"], ["0", "0"], ["0", "0"], ["0", "0"]]
  out "测试项目及频点在txt输出":string="$\nSDD21 TX1\n           RX1\n           TX2\n           RX2\n           TX3\n           RX3\n           TX4\n           RX4 #\nSDD11 TX1\n           RX1\n           TX2\n           RX2\n           TX3\n           RX3\n           TX4\n           RX4 #\nSCD22 TX1\n           RX1\n           TX2\n           RX2\n           TX3\n           RX3\n           TX4\n           RX4 #\nSCC11 TX1\n           RX1\n           TX2\n           RX2\n           TX3\n           RX3\n           TX4\n           RX4 #\nSCD21-SDD21 TX1\n           RX1\n           TX2\n           RX2\n           TX3\n           RX3\n           TX4\n           RX4 #\nILD_15 TX1\n           RX1\n           TX2\n           RX2\n           TX3\n           RX3\n           TX4\n           RX4 #$\n"